vi "run_pharmaBotExp_v0.015.vi"(0 "data in":T12={"daq_ao 1"="Dev1/ao0", "daq_ai 1"="Dev1/ai0", "experiment day folder"=path "C:/multiBot/data/debug/testing", "Multiclamp init error"=0, "Multiclamp Handle Out"=10225184, "sampling rate (Hz)"=20000, "trial name"="t1"}, 1 "auto run?":bool=TRUE, 3 "which manipulator":T13(ring), 4 "HEK/slice options":enum16{"slice", "HEK"}(ring), 5 "error in":errorcluster, 6 "Validate after Experiment":bool, 7 "common cluster":T9, 11 "individual controls in":T8, 13 "images":T3={"slice image"="remote image 000000001461186C", "pipette template"="remote image 000000001461152C", "found pipette"=refnum, "pipette mask for cell tracker"=refnum, "cell images ref"=refnum}) -> (10 "Cell Looks Good?":bool=TRUE, 12 "ValidationOutputCluster":T5(array[cluster]), 14 "ValidationResults":waveform(dbl)[][](array[waveform]), 15 "ValidationPos1":T6(array[ring]), 16 "Exp. Terminated":bool, 17 "ValidationPos2":T6(array[ring]), 18 "ValidationWaveform":waveform(dbl)[](array[waveform]), 19 "error out":errorcluster)   [LabVIEW 2015] (continued)
              frame "Gap Free Iclamp" {
                n1665 = property class="TabCtl (strict)"(reference=w2342, "Value"=w2341) -> ()  [unwired: 1 in, 2 out]
                n1666 = property class="TabCtl (strict)"(reference=w2342, "Visible"=TRUE) -> ()  [unwired: 1 in, 2 out]
              }
              frame "Current Pulse" {
                n1667 = property class="TabCtl (strict)"(reference=w2345, "Value"=w2344) -> ()  [unwired: 1 in, 2 out]
                n1668 = property class="TabCtl (strict)"(reference=w2345, "Visible"=TRUE) -> ()  [unwired: 1 in, 2 out]
              }
              frame "Current Ramp" {
                n1669 = property class="TabCtl (strict)"(reference=w2348, "Value"=w2347) -> ()  [unwired: 1 in, 2 out]
                n1670 = property class="TabCtl (strict)"(reference=w2348, "Visible"=TRUE) -> ()  [unwired: 1 in, 2 out]
              }
              frame "Multi M. Jump" {
                n1671 = property class="TabCtl (strict)"(reference=w2351, "Value"=w2350) -> ()  [unwired: 1 in, 2 out]
                n1672 = property class="TabCtl (strict)"(reference=w2351, "Visible"=TRUE) -> ()  [unwired: 1 in, 2 out]
              }
              frame "none" {
                n1673 = property class="TabCtl (strict)"(reference=w2353, "Visible"=FALSE) -> ()  [unwired: 1 in, 2 out]
              }
            }
          }
          frame "PhaseL Experiment Option" {
            n1674 = control-ref of="Experiment Selection L"() -> (w2368:refnum<vi>)
            n1675 = case shown="\"Current Ramp\"" w2369 {
              tunnel: w2368 -> [_ w2371 w2374 w2377 w2380 w2383 w2386 w2389 w2392 w2395 w2398 w2401 w2404 w2407 w2409]
              tunnel: w2367 -> [_ _ _ _ _ _ _ _ _ _ _ _ _ w2406 _]
              tunnel: w2366 -> [_ w2370 _ _ _ _ _ _ _ _ _ _ _ _ _]
              tunnel: w2365 -> [_ _ w2373 _ _ _ _ _ _ _ _ _ _ _ _]
              tunnel: w2364 -> [_ _ _ w2376 _ _ _ _ _ _ _ _ _ _ _]
              tunnel: w2363 -> [_ _ _ _ w2379 _ _ _ _ _ _ _ _ _ _]
              tunnel: w2362 -> [_ _ _ _ _ w2382 _ _ _ _ _ _ _ _ _]
              tunnel: w2361 -> [_ _ _ _ _ _ w2385 _ _ _ _ _ _ _ _]
              tunnel: w2360 -> [_ _ _ _ _ _ _ w2388 _ _ _ _ _ _ _]
              tunnel: w2359 -> [_ _ _ _ _ _ _ _ w2391 _ _ _ _ _ _]
              tunnel: w2358 -> [_ _ _ _ _ _ _ _ _ w2394 _ _ _ _ _]
              tunnel: w2357 -> [_ _ _ _ _ _ _ _ _ _ w2397 _ _ _ _]
              tunnel: w2356 -> [_ _ _ _ _ _ _ _ _ _ _ w2400 _ _ _]
              tunnel: w2355 -> [_ _ _ _ _ _ _ _ _ _ _ _ w2403 _ _]
              frame "False", Default {
              }
              frame "Single Jump" {
                n1676 = property class="TabCtl (strict)"(reference=w2371, "Value"=w2370) -> ()  [unwired: 1 in, 2 out]
                n1677 = property class="TabCtl (strict)"(reference=w2371, "Visible"=TRUE) -> ()  [unwired: 1 in, 2 out]
              }
              frame "Solution Change" {
                n1678 = property class="TabCtl (strict)"(reference=w2374, "Visible"=TRUE) -> ()  [unwired: 1 in, 2 out]
                n1679 = property class="TabCtl (strict)"(reference=w2374, "Value"=w2373) -> ()  [unwired: 1 in, 2 out]
              }
              frame "Voltage Step" {
                n1680 = property class="TabCtl (strict)"(reference=w2377, "Value"=w2376) -> ()  [unwired: 1 in, 2 out]
                n1681 = property class="TabCtl (strict)"(reference=w2377, "Visible"=TRUE) -> ()  [unwired: 1 in, 2 out]
              }
              frame "Voltage Ramp" {
                n1682 = property class="TabCtl (strict)"(reference=w2380, "Value"=w2379) -> ()  [unwired: 1 in, 2 out]
                n1683 = property class="TabCtl (strict)"(reference=w2380, "Visible"=TRUE) -> ()  [unwired: 1 in, 2 out]
              }
              frame "Voltage Pulse" {
                n1684 = property class="TabCtl (strict)"(reference=w2383, "Value"=w2382) -> ()  [unwired: 1 in, 2 out]
                n1685 = property class="TabCtl (strict)"(reference=w2383, "Visible"=TRUE) -> ()  [unwired: 1 in, 2 out]
              }
              frame "Jump Train" {
                n1686 = property class="TabCtl (strict)"(reference=w2386, "Value"=w2385) -> ()  [unwired: 1 in, 2 out]
                n1687 = property class="TabCtl (strict)"(reference=w2386, "Visible"=TRUE) -> ()  [unwired: 1 in, 2 out]
              }
              frame "Paired Pulse" {
                n1688 = property class="TabCtl (strict)"(reference=w2389, "Value"=w2388) -> ()  [unwired: 1 in, 2 out]
                n1689 = property class="TabCtl (strict)"(reference=w2389, "Visible"=TRUE) -> ()  [unwired: 1 in, 2 out]
              }
              frame "Single Manip Jump" {
                n1690 = property class="TabCtl (strict)"(reference=w2392, "Value"=w2391) -> ()  [unwired: 1 in, 2 out]
                n1691 = property class="TabCtl (strict)"(reference=w2392, "Visible"=TRUE) -> ()  [unwired: 1 in, 2 out]
              }
              frame "Gap Free" {
                n1692 = property class="TabCtl (strict)"(reference=w2395, "Value"=w2394) -> ()  [unwired: 1 in, 2 out]
                n1693 = property class="TabCtl (strict)"(reference=w2395, "Visible"=TRUE) -> ()  [unwired: 1 in, 2 out]
              }
              frame "Gap Free Iclamp" {
                n1694 = property class="TabCtl (strict)"(reference=w2398, "Value"=w2397) -> ()  [unwired: 1 in, 2 out]
                n1695 = property class="TabCtl (strict)"(reference=w2398, "Visible"=TRUE) -> ()  [unwired: 1 in, 2 out]
              }
              frame "Current Pulse" {
                n1696 = property class="TabCtl (strict)"(reference=w2401, "Value"=w2400) -> ()  [unwired: 1 in, 2 out]
                n1697 = property class="TabCtl (strict)"(reference=w2401, "Visible"=TRUE) -> ()  [unwired: 1 in, 2 out]
              }
              frame "Current Ramp" {
                n1698 = property class="TabCtl (strict)"(reference=w2404, "Value"=w2403) -> ()  [unwired: 1 in, 2 out]
                n1699 = property class="TabCtl (strict)"(reference=w2404, "Visible"=TRUE) -> ()  [unwired: 1 in, 2 out]
              }
              frame "Multi M. Jump" {
                n1700 = property class="TabCtl (strict)"(reference=w2407, "Value"=w2406) -> ()  [unwired: 1 in, 2 out]
                n1701 = property class="TabCtl (strict)"(reference=w2407, "Visible"=TRUE) -> ()  [unwired: 1 in, 2 out]
              }
              frame "none" {
                n1702 = property class="TabCtl (strict)"(reference=w2409, "Visible"=FALSE) -> ()  [unwired: 1 in, 2 out]
              }
            }
          }
        }
      }
      event "How Many Experimental Phases?": Value Change {
        n1703 = event-data() -> ("NewVal"=w2412:i32)  [unwired: 1 in, 5 out]
        n1704 = case shown="12" w2412 {
          frame 0, Default {
          }
          frame 1 {
            n1705 = control-ref of="PhaseB Experiment Option"() -> (w2458:refnum<vi>)
            n1706 = control-ref of="PhaseF Experiment Option"() -> (w2440:refnum<vi>)
            n1707 = control-ref of="PhaseA Experiment Option"() -> (w2460:refnum<vi>)
            n1708 = control-ref of="PhaseD Experiment Option"() -> (w2448:refnum<vi>)
            n1709 = control-ref of="PhaseC Experiment Option"() -> (w2449:refnum<vi>)
            n1710 = control-ref of="PhaseE Experiment Option"() -> (w2441:refnum<vi>)
            n1711 = property class="CmbBox"(reference=w2460, "Visible"=TRUE) -> ()  [unwired: 1 in, 2 out]
            n1712 = property class="CmbBox"(reference=w2458, "Visible"=FALSE) -> ()  [unwired: 1 in, 2 out]
            n1713 = property class="CmbBox"(reference=w2440, "Visible"=FALSE) -> ()  [unwired: 1 in, 2 out]
            n1714 = property class="CmbBox"(reference=w2448, "Visible"=FALSE) -> ()  [unwired: 1 in, 2 out]
            n1715 = property class="CmbBox"(reference=w2449, "Visible"=FALSE) -> ()  [unwired: 1 in, 2 out]
            n1716 = property class="CmbBox"(reference=w2441, "Visible"=FALSE) -> ()  [unwired: 1 in, 2 out]
            n1717 = control-ref of="Experiment Selection B"() -> (w2455:refnum<vi>)
            n1718 = control-ref of="Experiment Selection F"() -> (w2437:refnum<vi>)
            n1719 = control-ref of="Experiment Selection D"() -> (w2445:refnum<vi>)
            n1720 = control-ref of="Experiment Selection A"() -> (w2453:refnum<vi>)
            n1721 = control-ref of="Experiment Selection C"() -> (w2452:refnum<vi>)
            n1722 = control-ref of="Experiment Selection E"() -> (w2444:refnum<vi>)
            n1723 = property class="TabCtl (strict)"(reference=w2455, "Visible"=FALSE) -> ()  [unwired: 1 in, 2 out]
            n1724 = property class="TabCtl (strict)"(reference=w2453, "Visible"=TRUE) -> ()  [unwired: 1 in, 2 out]
            n1725 = property class="TabCtl (strict)"(reference=w2437, "Visible"=FALSE) -> ()  [unwired: 1 in, 2 out]
            n1726 = property class="TabCtl (strict)"(reference=w2445, "Visible"=FALSE) -> ()  [unwired: 1 in, 2 out]
            n1727 = property class="TabCtl (strict)"(reference=w2452, "Visible"=FALSE) -> ()  [unwired: 1 in, 2 out]
            n1728 = property class="TabCtl (strict)"(reference=w2444, "Visible"=FALSE) -> ()  [unwired: 1 in, 2 out]
            n1729 = control-ref of="PhaseH Experiment Option"() -> (w2415:refnum<vi>)
            n1730 = control-ref of="PhaseL Experiment Option"() -> (w2433:refnum<vi>)
            n1731 = control-ref of="PhaseG Experiment Option"() -> (w2413:refnum<vi>)
            n1732 = control-ref of="PhaseJ Experiment Option"() -> (w2425:refnum<vi>)
            n1733 = control-ref of="PhaseI Experiment Option"() -> (w2424:refnum<vi>)
            n1734 = control-ref of="PhaseK Experiment Option"() -> (w2432:refnum<vi>)
            n1735 = property class="CmbBox"(reference=w2413, "Visible"=FALSE) -> ()  [unwired: 1 in, 2 out]
            n1736 = property class="CmbBox"(reference=w2415, "Visible"=FALSE) -> ()  [unwired: 1 in, 2 out]
            n1737 = property class="CmbBox"(reference=w2433, "Visible"=FALSE) -> ()  [unwired: 1 in, 2 out]
            n1738 = property class="CmbBox"(reference=w2425, "Visible"=FALSE) -> ()  [unwired: 1 in, 2 out]
            n1739 = property class="CmbBox"(reference=w2424, "Visible"=FALSE) -> ()  [unwired: 1 in, 2 out]
            n1740 = property class="CmbBox"(reference=w2432, "Visible"=FALSE) -> ()  [unwired: 1 in, 2 out]
            n1741 = control-ref of="Experiment Selection H"() -> (w2418:refnum<vi>)
            n1742 = control-ref of="Experiment Selection L"() -> (w2436:refnum<vi>)
            n1743 = control-ref of="Experiment Selection J"() -> (w2428:refnum<vi>)
            n1744 = control-ref of="Experiment Selection G"() -> (w2420:refnum<vi>)
            n1745 = control-ref of="Experiment Selection I"() -> (w2421:refnum<vi>)
            n1746 = control-ref of="Experiment Selection K"() -> (w2429:refnum<vi>)
            n1747 = property class="TabCtl (strict)"(reference=w2418, "Visible"=FALSE) -> ()  [unwired: 1 in, 2 out]
            n1748 = property class="TabCtl (strict)"(reference=w2420, "Visible"=FALSE) -> ()  [unwired: 1 in, 2 out]
            n1749 = property class="TabCtl (strict)"(reference=w2436, "Visible"=FALSE) -> ()  [unwired: 1 in, 2 out]
            n1750 = property class="TabCtl (strict)"(reference=w2428, "Visible"=FALSE) -> ()  [unwired: 1 in, 2 out]
            n1751 = property class="TabCtl (strict)"(reference=w2421, "Visible"=FALSE) -> ()  [unwired: 1 in, 2 out]
            n1752 = property class="TabCtl (strict)"(reference=w2429, "Visible"=FALSE) -> ()  [unwired: 1 in, 2 out]
          }
          frame 2 {
            n1753 = control-ref of="PhaseB Experiment Option"() -> (w2506:refnum<vi>)
            n1754 = control-ref of="PhaseF Experiment Option"() -> (w2488:refnum<vi>)
            n1755 = control-ref of="PhaseA Experiment Option"() -> (w2508:refnum<vi>)
            n1756 = control-ref of="PhaseD Experiment Option"() -> (w2496:refnum<vi>)
            n1757 = control-ref of="PhaseC Experiment Option"() -> (w2497:refnum<vi>)
            n1758 = control-ref of="PhaseE Experiment Option"() -> (w2489:refnum<vi>)
            n1759 = property class="CmbBox"(reference=w2508, "Visible"=TRUE) -> ()  [unwired: 1 in, 2 out]
            n1760 = property class="CmbBox"(reference=w2506, "Visible"=TRUE) -> ()  [unwired: 1 in, 2 out]
            n1761 = property class="CmbBox"(reference=w2488, "Visible"=FALSE) -> ()  [unwired: 1 in, 2 out]
            n1762 = property class="CmbBox"(reference=w2496, "Visible"=FALSE) -> ()  [unwired: 1 in, 2 out]
            n1763 = property class="CmbBox"(reference=w2497, "Visible"=FALSE) -> ()  [unwired: 1 in, 2 out]
            n1764 = property class="CmbBox"(reference=w2489, "Visible"=FALSE) -> ()  [unwired: 1 in, 2 out]
            n1765 = control-ref of="Experiment Selection B"() -> (w2503:refnum<vi>)
            n1766 = control-ref of="Experiment Selection F"() -> (w2485:refnum<vi>)
            n1767 = control-ref of="Experiment Selection D"() -> (w2493:refnum<vi>)
            n1768 = control-ref of="Experiment Selection A"() -> (w2501:refnum<vi>)
            n1769 = control-ref of="Experiment Selection C"() -> (w2500:refnum<vi>)
            n1770 = control-ref of="Experiment Selection E"() -> (w2492:refnum<vi>)
            n1771 = property class="TabCtl (strict)"(reference=w2503, "Visible"=TRUE) -> ()  [unwired: 1 in, 2 out]
            n1772 = property class="TabCtl (strict)"(reference=w2501, "Visible"=TRUE) -> ()  [unwired: 1 in, 2 out]
            n1773 = property class="TabCtl (strict)"(reference=w2485, "Visible"=FALSE) -> ()  [unwired: 1 in, 2 out]
            n1774 = property class="TabCtl (strict)"(reference=w2493, "Visible"=FALSE) -> ()  [unwired: 1 in, 2 out]
            n1775 = property class="TabCtl (strict)"(reference=w2500, "Visible"=FALSE) -> ()  [unwired: 1 in, 2 out]
            n1776 = property class="TabCtl (strict)"(reference=w2492, "Visible"=FALSE) -> ()  [unwired: 1 in, 2 out]
            n1777 = control-ref of="PhaseH Experiment Option"() -> (w2463:refnum<vi>)
            n1778 = control-ref of="PhaseL Experiment Option"() -> (w2481:refnum<vi>)
            n1779 = control-ref of="PhaseG Experiment Option"() -> (w2461:refnum<vi>)
            n1780 = control-ref of="PhaseJ Experiment Option"() -> (w2473:refnum<vi>)
            n1781 = control-ref of="PhaseI Experiment Option"() -> (w2472:refnum<vi>)
            n1782 = control-ref of="PhaseK Experiment Option"() -> (w2480:refnum<vi>)
            n1783 = property class="CmbBox"(reference=w2461, "Visible"=FALSE) -> ()  [unwired: 1 in, 2 out]
            n1784 = property class="CmbBox"(reference=w2463, "Visible"=FALSE) -> ()  [unwired: 1 in, 2 out]
            n1785 = property class="CmbBox"(reference=w2481, "Visible"=FALSE) -> ()  [unwired: 1 in, 2 out]
            n1786 = property class="CmbBox"(reference=w2473, "Visible"=FALSE) -> ()  [unwired: 1 in, 2 out]
            n1787 = property class="CmbBox"(reference=w2472, "Visible"=FALSE) -> ()  [unwired: 1 in, 2 out]
            n1788 = property class="CmbBox"(reference=w2480, "Visible"=FALSE) -> ()  [unwired: 1 in, 2 out]
            n1789 = control-ref of="Experiment Selection H"() -> (w2466:refnum<vi>)
            n1790 = control-ref of="Experiment Selection L"() -> (w2484:refnum<vi>)
            n1791 = control-ref of="Experiment Selection J"() -> (w2476:refnum<vi>)
            n1792 = control-ref of="Experiment Selection G"() -> (w2468:refnum<vi>)
            n1793 = control-ref of="Experiment Selection I"() -> (w2469:refnum<vi>)
            n1794 = control-ref of="Experiment Selection K"() -> (w2477:refnum<vi>)
            n1795 = property class="TabCtl (strict)"(reference=w2466, "Visible"=FALSE) -> ()  [unwired: 1 in, 2 out]
            n1796 = property class="TabCtl (strict)"(reference=w2468, "Visible"=FALSE) -> ()  [unwired: 1 in, 2 out]
            n1797 = property class="TabCtl (strict)"(reference=w2484, "Visible"=FALSE) -> ()  [unwired: 1 in, 2 out]
            n1798 = property class="TabCtl (strict)"(reference=w2476, "Visible"=FALSE) -> ()  [unwired: 1 in, 2 out]
            n1799 = property class="TabCtl (strict)"(reference=w2469, "Visible"=FALSE) -> ()  [unwired: 1 in, 2 out]
            n1800 = property class="TabCtl (strict)"(reference=w2477, "Visible"=FALSE) -> ()  [unwired: 1 in, 2 out]
          }
          frame 3 {
            n1801 = control-ref of="PhaseB Experiment Option"() -> (w2554:refnum<vi>)
            n1802 = control-ref of="PhaseF Experiment Option"() -> (w2536:refnum<vi>)
            n1803 = control-ref of="PhaseA Experiment Option"() -> (w2556:refnum<vi>)
            n1804 = control-ref of="PhaseD Experiment Option"() -> (w2544:refnum<vi>)
            n1805 = control-ref of="PhaseC Experiment Option"() -> (w2545:refnum<vi>)
            n1806 = control-ref of="PhaseE Experiment Option"() -> (w2537:refnum<vi>)
            n1807 = property class="CmbBox"(reference=w2556, "Visible"=TRUE) -> ()  [unwired: 1 in, 2 out]
            n1808 = property class="CmbBox"(reference=w2554, "Visible"=TRUE) -> ()  [unwired: 1 in, 2 out]
            n1809 = property class="CmbBox"(reference=w2536, "Visible"=FALSE) -> ()  [unwired: 1 in, 2 out]
            n1810 = property class="CmbBox"(reference=w2544, "Visible"=FALSE) -> ()  [unwired: 1 in, 2 out]
            n1811 = property class="CmbBox"(reference=w2545, "Visible"=TRUE) -> ()  [unwired: 1 in, 2 out]
            n1812 = property class="CmbBox"(reference=w2537, "Visible"=FALSE) -> ()  [unwired: 1 in, 2 out]
            n1813 = control-ref of="Experiment Selection B"() -> (w2551:refnum<vi>)
            n1814 = control-ref of="Experiment Selection F"() -> (w2533:refnum<vi>)
            n1815 = control-ref of="Experiment Selection D"() -> (w2541:refnum<vi>)
            n1816 = control-ref of="Experiment Selection A"() -> (w2549:refnum<vi>)
            n1817 = control-ref of="Experiment Selection C"() -> (w2548:refnum<vi>)
            n1818 = control-ref of="Experiment Selection E"() -> (w2540:refnum<vi>)
            n1819 = property class="TabCtl (strict)"(reference=w2551, "Visible"=TRUE) -> ()  [unwired: 1 in, 2 out]
            n1820 = property class="TabCtl (strict)"(reference=w2549, "Visible"=TRUE) -> ()  [unwired: 1 in, 2 out]
            n1821 = property class="TabCtl (strict)"(reference=w2533, "Visible"=FALSE) -> ()  [unwired: 1 in, 2 out]
            n1822 = property class="TabCtl (strict)"(reference=w2541, "Visible"=FALSE) -> ()  [unwired: 1 in, 2 out]
            n1823 = property class="TabCtl (strict)"(reference=w2548, "Visible"=TRUE) -> ()  [unwired: 1 in, 2 out]
            n1824 = property class="TabCtl (strict)"(reference=w2540, "Visible"=FALSE) -> ()  [unwired: 1 in, 2 out]
            n1825 = control-ref of="PhaseH Experiment Option"() -> (w2511:refnum<vi>)
            n1826 = control-ref of="PhaseL Experiment Option"() -> (w2529:refnum<vi>)
            n1827 = control-ref of="PhaseG Experiment Option"() -> (w2509:refnum<vi>)
            n1828 = control-ref of="PhaseJ Experiment Option"() -> (w2521:refnum<vi>)
            n1829 = control-ref of="PhaseI Experiment Option"() -> (w2520:refnum<vi>)
            n1830 = control-ref of="PhaseK Experiment Option"() -> (w2528:refnum<vi>)
            n1831 = property class="CmbBox"(reference=w2509, "Visible"=FALSE) -> ()  [unwired: 1 in, 2 out]
            n1832 = property class="CmbBox"(reference=w2511, "Visible"=FALSE) -> ()  [unwired: 1 in, 2 out]
            n1833 = property class="CmbBox"(reference=w2529, "Visible"=FALSE) -> ()  [unwired: 1 in, 2 out]
            n1834 = property class="CmbBox"(reference=w2521, "Visible"=FALSE) -> ()  [unwired: 1 in, 2 out]
            n1835 = property class="CmbBox"(reference=w2520, "Visible"=FALSE) -> ()  [unwired: 1 in, 2 out]
            n1836 = property class="CmbBox"(reference=w2528, "Visible"=FALSE) -> ()  [unwired: 1 in, 2 out]
            n1837 = control-ref of="Experiment Selection H"() -> (w2514:refnum<vi>)
            n1838 = control-ref of="Experiment Selection L"() -> (w2532:refnum<vi>)
            n1839 = control-ref of="Experiment Selection J"() -> (w2524:refnum<vi>)
            n1840 = control-ref of="Experiment Selection G"() -> (w2516:refnum<vi>)
            n1841 = control-ref of="Experiment Selection I"() -> (w2517:refnum<vi>)
            n1842 = control-ref of="Experiment Selection K"() -> (w2525:refnum<vi>)
            n1843 = property class="TabCtl (strict)"(reference=w2514, "Visible"=FALSE) -> ()  [unwired: 1 in, 2 out]
            n1844 = property class="TabCtl (strict)"(reference=w2516, "Visible"=FALSE) -> ()  [unwired: 1 in, 2 out]
            n1845 = property class="TabCtl (strict)"(reference=w2532, "Visible"=FALSE) -> ()  [unwired: 1 in, 2 out]
            n1846 = property class="TabCtl (strict)"(reference=w2524, "Visible"=FALSE) -> ()  [unwired: 1 in, 2 out]
            n1847 = property class="TabCtl (strict)"(reference=w2517, "Visible"=FALSE) -> ()  [unwired: 1 in, 2 out]
            n1848 = property class="TabCtl (strict)"(reference=w2525, "Visible"=FALSE) -> ()  [unwired: 1 in, 2 out]
          }
          frame 4 {
            n1849 = control-ref of="PhaseB Experiment Option"() -> (w2602:refnum<vi>)
            n1850 = control-ref of="PhaseF Experiment Option"() -> (w2584:refnum<vi>)
            n1851 = control-ref of="PhaseA Experiment Option"() -> (w2604:refnum<vi>)
            n1852 = control-ref of="PhaseD Experiment Option"() -> (w2592:refnum<vi>)
            n1853 = control-ref of="PhaseC Experiment Option"() -> (w2593:refnum<vi>)
            n1854 = control-ref of="PhaseE Experiment Option"() -> (w2585:refnum<vi>)
            n1855 = property class="CmbBox"(reference=w2604, "Visible"=TRUE) -> ()  [unwired: 1 in, 2 out]
            n1856 = property class="CmbBox"(reference=w2602, "Visible"=TRUE) -> ()  [unwired: 1 in, 2 out]
            n1857 = property class="CmbBox"(reference=w2584, "Visible"=FALSE) -> ()  [unwired: 1 in, 2 out]
            n1858 = property class="CmbBox"(reference=w2592, "Visible"=TRUE) -> ()  [unwired: 1 in, 2 out]
            n1859 = property class="CmbBox"(reference=w2593, "Visible"=TRUE) -> ()  [unwired: 1 in, 2 out]
            n1860 = property class="CmbBox"(reference=w2585, "Visible"=FALSE) -> ()  [unwired: 1 in, 2 out]
            n1861 = control-ref of="Experiment Selection B"() -> (w2599:refnum<vi>)
            n1862 = control-ref of="Experiment Selection F"() -> (w2581:refnum<vi>)
            n1863 = control-ref of="Experiment Selection D"() -> (w2589:refnum<vi>)
            n1864 = control-ref of="Experiment Selection A"() -> (w2597:refnum<vi>)
            n1865 = control-ref of="Experiment Selection C"() -> (w2596:refnum<vi>)
            n1866 = control-ref of="Experiment Selection E"() -> (w2588:refnum<vi>)
            n1867 = property class="TabCtl (strict)"(reference=w2599, "Visible"=TRUE) -> ()  [unwired: 1 in, 2 out]
            n1868 = property class="TabCtl (strict)"(reference=w2597, "Visible"=TRUE) -> ()  [unwired: 1 in, 2 out]
            n1869 = property class="TabCtl (strict)"(reference=w2581, "Visible"=FALSE) -> ()  [unwired: 1 in, 2 out]
            n1870 = property class="TabCtl (strict)"(reference=w2589, "Visible"=TRUE) -> ()  [unwired: 1 in, 2 out]
            n1871 = property class="TabCtl (strict)"(reference=w2596, "Visible"=TRUE) -> ()  [unwired: 1 in, 2 out]
            n1872 = property class="TabCtl (strict)"(reference=w2588, "Visible"=FALSE) -> ()  [unwired: 1 in, 2 out]
            n1873 = control-ref of="PhaseH Experiment Option"() -> (w2559:refnum<vi>)
            n1874 = control-ref of="PhaseL Experiment Option"() -> (w2577:refnum<vi>)
            n1875 = control-ref of="PhaseG Experiment Option"() -> (w2557:refnum<vi>)
            n1876 = control-ref of="PhaseJ Experiment Option"() -> (w2569:refnum<vi>)
            n1877 = control-ref of="PhaseI Experiment Option"() -> (w2568:refnum<vi>)
            n1878 = control-ref of="PhaseK Experiment Option"() -> (w2576:refnum<vi>)
            n1879 = property class="CmbBox"(reference=w2557, "Visible"=FALSE) -> ()  [unwired: 1 in, 2 out]
            n1880 = property class="CmbBox"(reference=w2559, "Visible"=FALSE) -> ()  [unwired: 1 in, 2 out]
            n1881 = property class="CmbBox"(reference=w2577, "Visible"=FALSE) -> ()  [unwired: 1 in, 2 out]
            n1882 = property class="CmbBox"(reference=w2569, "Visible"=FALSE) -> ()  [unwired: 1 in, 2 out]
            n1883 = property class="CmbBox"(reference=w2568, "Visible"=FALSE) -> ()  [unwired: 1 in, 2 out]
            n1884 = property class="CmbBox"(reference=w2576, "Visible"=FALSE) -> ()  [unwired: 1 in, 2 out]
            n1885 = control-ref of="Experiment Selection H"() -> (w2562:refnum<vi>)
            n1886 = control-ref of="Experiment Selection L"() -> (w2580:refnum<vi>)
            n1887 = control-ref of="Experiment Selection J"() -> (w2572:refnum<vi>)
            n1888 = control-ref of="Experiment Selection G"() -> (w2564:refnum<vi>)
            n1889 = control-ref of="Experiment Selection I"() -> (w2565:refnum<vi>)
            n1890 = control-ref of="Experiment Selection K"() -> (w2573:refnum<vi>)
            n1891 = property class="TabCtl (strict)"(reference=w2562, "Visible"=FALSE) -> ()  [unwired: 1 in, 2 out]
            n1892 = property class="TabCtl (strict)"(reference=w2564, "Visible"=FALSE) -> ()  [unwired: 1 in, 2 out]
            n1893 = property class="TabCtl (strict)"(reference=w2580, "Visible"=FALSE) -> ()  [unwired: 1 in, 2 out]
            n1894 = property class="TabCtl (strict)"(reference=w2572, "Visible"=FALSE) -> ()  [unwired: 1 in, 2 out]
            n1895 = property class="TabCtl (strict)"(reference=w2565, "Visible"=FALSE) -> ()  [unwired: 1 in, 2 out]
            n1896 = property class="TabCtl (strict)"(reference=w2573, "Visible"=FALSE) -> ()  [unwired: 1 in, 2 out]
          }
          frame 5 {
            n1897 = control-ref of="PhaseB Experiment Option"() -> (w2650:refnum<vi>)
            n1898 = control-ref of="PhaseF Experiment Option"() -> (w2632:refnum<vi>)
            n1899 = control-ref of="PhaseA Experiment Option"() -> (w2652:refnum<vi>)
            n1900 = control-ref of="PhaseD Experiment Option"() -> (w2640:refnum<vi>)
            n1901 = control-ref of="PhaseC Experiment Option"() -> (w2641:refnum<vi>)
            n1902 = control-ref of="PhaseE Experiment Option"() -> (w2633:refnum<vi>)
            n1903 = property class="CmbBox"(reference=w2652, "Visible"=TRUE) -> ()  [unwired: 1 in, 2 out]
            n1904 = property class="CmbBox"(reference=w2650, "Visible"=TRUE) -> ()  [unwired: 1 in, 2 out]
            n1905 = property class="CmbBox"(reference=w2632, "Visible"=FALSE) -> ()  [unwired: 1 in, 2 out]
            n1906 = property class="CmbBox"(reference=w2640, "Visible"=TRUE) -> ()  [unwired: 1 in, 2 out]
            n1907 = property class="CmbBox"(reference=w2641, "Visible"=TRUE) -> ()  [unwired: 1 in, 2 out]
            n1908 = property class="CmbBox"(reference=w2633, "Visible"=TRUE) -> ()  [unwired: 1 in, 2 out]
            n1909 = control-ref of="Experiment Selection B"() -> (w2647:refnum<vi>)
            n1910 = control-ref of="Experiment Selection F"() -> (w2629:refnum<vi>)
            n1911 = control-ref of="Experiment Selection D"() -> (w2637:refnum<vi>)
            n1912 = control-ref of="Experiment Selection A"() -> (w2645:refnum<vi>)
            n1913 = control-ref of="Experiment Selection C"() -> (w2644:refnum<vi>)
            n1914 = control-ref of="Experiment Selection E"() -> (w2636:refnum<vi>)
            n1915 = property class="TabCtl (strict)"(reference=w2647, "Visible"=TRUE) -> ()  [unwired: 1 in, 2 out]
            n1916 = property class="TabCtl (strict)"(reference=w2645, "Visible"=TRUE) -> ()  [unwired: 1 in, 2 out]
            n1917 = property class="TabCtl (strict)"(reference=w2629, "Visible"=FALSE) -> ()  [unwired: 1 in, 2 out]
            n1918 = property class="TabCtl (strict)"(reference=w2637, "Visible"=TRUE) -> ()  [unwired: 1 in, 2 out]
            n1919 = property class="TabCtl (strict)"(reference=w2644, "Visible"=TRUE) -> ()  [unwired: 1 in, 2 out]
            n1920 = property class="TabCtl (strict)"(reference=w2636, "Visible"=TRUE) -> ()  [unwired: 1 in, 2 out]
            n1921 = control-ref of="PhaseH Experiment Option"() -> (w2607:refnum<vi>)
            n1922 = control-ref of="PhaseL Experiment Option"() -> (w2625:refnum<vi>)
            n1923 = control-ref of="PhaseG Experiment Option"() -> (w2605:refnum<vi>)
            n1924 = control-ref of="PhaseJ Experiment Option"() -> (w2617:refnum<vi>)
            n1925 = control-ref of="PhaseI Experiment Option"() -> (w2616:refnum<vi>)
            n1926 = control-ref of="PhaseK Experiment Option"() -> (w2624:refnum<vi>)
            n1927 = property class="CmbBox"(reference=w2605, "Visible"=FALSE) -> ()  [unwired: 1 in, 2 out]
            n1928 = property class="CmbBox"(reference=w2607, "Visible"=FALSE) -> ()  [unwired: 1 in, 2 out]
            n1929 = property class="CmbBox"(reference=w2625, "Visible"=FALSE) -> ()  [unwired: 1 in, 2 out]
            n1930 = property class="CmbBox"(reference=w2617, "Visible"=FALSE) -> ()  [unwired: 1 in, 2 out]
            n1931 = property class="CmbBox"(reference=w2616, "Visible"=FALSE) -> ()  [unwired: 1 in, 2 out]
            n1932 = property class="CmbBox"(reference=w2624, "Visible"=FALSE) -> ()  [unwired: 1 in, 2 out]
            n1933 = control-ref of="Experiment Selection H"() -> (w2610:refnum<vi>)
            n1934 = control-ref of="Experiment Selection L"() -> (w2628:refnum<vi>)
            n1935 = control-ref of="Experiment Selection J"() -> (w2620:refnum<vi>)
            n1936 = control-ref of="Experiment Selection G"() -> (w2612:refnum<vi>)
            n1937 = control-ref of="Experiment Selection I"() -> (w2613:refnum<vi>)
            n1938 = control-ref of="Experiment Selection K"() -> (w2621:refnum<vi>)
            n1939 = property class="TabCtl (strict)"(reference=w2610, "Visible"=FALSE) -> ()  [unwired: 1 in, 2 out]
            n1940 = property class="TabCtl (strict)"(reference=w2612, "Visible"=FALSE) -> ()  [unwired: 1 in, 2 out]
            n1941 = property class="TabCtl (strict)"(reference=w2628, "Visible"=FALSE) -> ()  [unwired: 1 in, 2 out]
            n1942 = property class="TabCtl (strict)"(reference=w2620, "Visible"=FALSE) -> ()  [unwired: 1 in, 2 out]
            n1943 = property class="TabCtl (strict)"(reference=w2613, "Visible"=FALSE) -> ()  [unwired: 1 in, 2 out]
            n1944 = property class="TabCtl (strict)"(reference=w2621, "Visible"=FALSE) -> ()  [unwired: 1 in, 2 out]
          }
          frame 6 {
            n1945 = control-ref of="PhaseB Experiment Option"() -> (w2698:refnum<vi>)
            n1946 = control-ref of="PhaseF Experiment Option"() -> (w2680:refnum<vi>)
            n1947 = control-ref of="PhaseA Experiment Option"() -> (w2700:refnum<vi>)
            n1948 = control-ref of="PhaseD Experiment Option"() -> (w2688:refnum<vi>)
            n1949 = control-ref of="PhaseC Experiment Option"() -> (w2689:refnum<vi>)
            n1950 = control-ref of="PhaseE Experiment Option"() -> (w2681:refnum<vi>)
            n1951 = property class="CmbBox"(reference=w2700, "Visible"=TRUE) -> ()  [unwired: 1 in, 2 out]
            n1952 = property class="CmbBox"(reference=w2698, "Visible"=TRUE) -> ()  [unwired: 1 in, 2 out]
            n1953 = property class="CmbBox"(reference=w2680, "Visible"=TRUE) -> ()  [unwired: 1 in, 2 out]
            n1954 = property class="CmbBox"(reference=w2688, "Visible"=TRUE) -> ()  [unwired: 1 in, 2 out]
            n1955 = property class="CmbBox"(reference=w2689, "Visible"=TRUE) -> ()  [unwired: 1 in, 2 out]
            n1956 = property class="CmbBox"(reference=w2681, "Visible"=TRUE) -> ()  [unwired: 1 in, 2 out]
            n1957 = control-ref of="Experiment Selection B"() -> (w2695:refnum<vi>)
            n1958 = control-ref of="Experiment Selection F"() -> (w2677:refnum<vi>)
            n1959 = control-ref of="Experiment Selection D"() -> (w2685:refnum<vi>)
            n1960 = control-ref of="Experiment Selection A"() -> (w2693:refnum<vi>)
            n1961 = control-ref of="Experiment Selection C"() -> (w2692:refnum<vi>)
            n1962 = control-ref of="Experiment Selection E"() -> (w2684:refnum<vi>)
            n1963 = property class="TabCtl (strict)"(reference=w2695, "Visible"=TRUE) -> ()  [unwired: 1 in, 2 out]
            n1964 = property class="TabCtl (strict)"(reference=w2693, "Visible"=TRUE) -> ()  [unwired: 1 in, 2 out]
            n1965 = property class="TabCtl (strict)"(reference=w2677, "Visible"=TRUE) -> ()  [unwired: 1 in, 2 out]
            n1966 = property class="TabCtl (strict)"(reference=w2685, "Visible"=TRUE) -> ()  [unwired: 1 in, 2 out]
            n1967 = property class="TabCtl (strict)"(reference=w2692, "Visible"=TRUE) -> ()  [unwired: 1 in, 2 out]
            n1968 = property class="TabCtl (strict)"(reference=w2684, "Visible"=TRUE) -> ()  [unwired: 1 in, 2 out]
            n1969 = control-ref of="PhaseH Experiment Option"() -> (w2655:refnum<vi>)
            n1970 = control-ref of="PhaseL Experiment Option"() -> (w2673:refnum<vi>)
            n1971 = control-ref of="PhaseG Experiment Option"() -> (w2653:refnum<vi>)
            n1972 = control-ref of="PhaseJ Experiment Option"() -> (w2665:refnum<vi>)
            n1973 = control-ref of="PhaseI Experiment Option"() -> (w2664:refnum<vi>)
            n1974 = control-ref of="PhaseK Experiment Option"() -> (w2672:refnum<vi>)
            n1975 = property class="CmbBox"(reference=w2653, "Visible"=FALSE) -> ()  [unwired: 1 in, 2 out]
            n1976 = property class="CmbBox"(reference=w2655, "Visible"=FALSE) -> ()  [unwired: 1 in, 2 out]
            n1977 = property class="CmbBox"(reference=w2673, "Visible"=FALSE) -> ()  [unwired: 1 in, 2 out]
            n1978 = property class="CmbBox"(reference=w2665, "Visible"=FALSE) -> ()  [unwired: 1 in, 2 out]
            n1979 = property class="CmbBox"(reference=w2664, "Visible"=FALSE) -> ()  [unwired: 1 in, 2 out]
            n1980 = property class="CmbBox"(reference=w2672, "Visible"=FALSE) -> ()  [unwired: 1 in, 2 out]
            n1981 = control-ref of="Experiment Selection H"() -> (w2658:refnum<vi>)
            n1982 = control-ref of="Experiment Selection L"() -> (w2676:refnum<vi>)
            n1983 = control-ref of="Experiment Selection J"() -> (w2668:refnum<vi>)
            n1984 = control-ref of="Experiment Selection G"() -> (w2660:refnum<vi>)
            n1985 = control-ref of="Experiment Selection I"() -> (w2661:refnum<vi>)
            n1986 = control-ref of="Experiment Selection K"() -> (w2669:refnum<vi>)
            n1987 = property class="TabCtl (strict)"(reference=w2658, "Visible"=FALSE) -> ()  [unwired: 1 in, 2 out]
            n1988 = property class="TabCtl (strict)"(reference=w2660, "Visible"=FALSE) -> ()  [unwired: 1 in, 2 out]
            n1989 = property class="TabCtl (strict)"(reference=w2676, "Visible"=FALSE) -> ()  [unwired: 1 in, 2 out]
            n1990 = property class="TabCtl (strict)"(reference=w2668, "Visible"=FALSE) -> ()  [unwired: 1 in, 2 out]
            n1991 = property class="TabCtl (strict)"(reference=w2661, "Visible"=FALSE) -> ()  [unwired: 1 in, 2 out]
            n1992 = property class="TabCtl (strict)"(reference=w2669, "Visible"=FALSE) -> ()  [unwired: 1 in, 2 out]
          }
          frame 7 {
            n1993 = control-ref of="PhaseB Experiment Option"() -> (w2746:refnum<vi>)
            n1994 = control-ref of="PhaseF Experiment Option"() -> (w2728:refnum<vi>)
            n1995 = control-ref of="PhaseA Experiment Option"() -> (w2748:refnum<vi>)
            n1996 = control-ref of="PhaseD Experiment Option"() -> (w2736:refnum<vi>)
            n1997 = control-ref of="PhaseC Experiment Option"() -> (w2737:refnum<vi>)
            n1998 = control-ref of="PhaseE Experiment Option"() -> (w2729:refnum<vi>)
            n1999 = property class="CmbBox"(reference=w2748, "Visible"=TRUE) -> ()  [unwired: 1 in, 2 out]
            n2000 = property class="CmbBox"(reference=w2746, "Visible"=TRUE) -> ()  [unwired: 1 in, 2 out]
            n2001 = property class="CmbBox"(reference=w2728, "Visible"=TRUE) -> ()  [unwired: 1 in, 2 out]
            n2002 = property class="CmbBox"(reference=w2736, "Visible"=TRUE) -> ()  [unwired: 1 in, 2 out]
            n2003 = property class="CmbBox"(reference=w2737, "Visible"=TRUE) -> ()  [unwired: 1 in, 2 out]
            n2004 = property class="CmbBox"(reference=w2729, "Visible"=TRUE) -> ()  [unwired: 1 in, 2 out]
            n2005 = control-ref of="Experiment Selection B"() -> (w2743:refnum<vi>)
            n2006 = control-ref of="Experiment Selection F"() -> (w2725:refnum<vi>)
            n2007 = control-ref of="Experiment Selection D"() -> (w2733:refnum<vi>)
            n2008 = control-ref of="Experiment Selection A"() -> (w2741:refnum<vi>)
            n2009 = control-ref of="Experiment Selection C"() -> (w2740:refnum<vi>)
            n2010 = control-ref of="Experiment Selection E"() -> (w2732:refnum<vi>)
            n2011 = property class="TabCtl (strict)"(reference=w2743, "Visible"=TRUE) -> ()  [unwired: 1 in, 2 out]
            n2012 = property class="TabCtl (strict)"(reference=w2741, "Visible"=TRUE) -> ()  [unwired: 1 in, 2 out]
            n2013 = property class="TabCtl (strict)"(reference=w2725, "Visible"=TRUE) -> ()  [unwired: 1 in, 2 out]
            n2014 = property class="TabCtl (strict)"(reference=w2733, "Visible"=TRUE) -> ()  [unwired: 1 in, 2 out]
            n2015 = property class="TabCtl (strict)"(reference=w2740, "Visible"=TRUE) -> ()  [unwired: 1 in, 2 out]
            n2016 = property class="TabCtl (strict)"(reference=w2732, "Visible"=TRUE) -> ()  [unwired: 1 in, 2 out]
            n2017 = control-ref of="PhaseH Experiment Option"() -> (w2703:refnum<vi>)
            n2018 = control-ref of="PhaseL Experiment Option"() -> (w2721:refnum<vi>)
            n2019 = control-ref of="PhaseG Experiment Option"() -> (w2701:refnum<vi>)
            n2020 = control-ref of="PhaseJ Experiment Option"() -> (w2713:refnum<vi>)
            n2021 = control-ref of="PhaseI Experiment Option"() -> (w2712:refnum<vi>)
            n2022 = control-ref of="PhaseK Experiment Option"() -> (w2720:refnum<vi>)
            n2023 = property class="CmbBox"(reference=w2701, "Visible"=TRUE) -> ()  [unwired: 1 in, 2 out]
            n2024 = property class="CmbBox"(reference=w2703, "Visible"=FALSE) -> ()  [unwired: 1 in, 2 out]
            n2025 = property class="CmbBox"(reference=w2721, "Visible"=FALSE) -> ()  [unwired: 1 in, 2 out]
            n2026 = property class="CmbBox"(reference=w2713, "Visible"=FALSE) -> ()  [unwired: 1 in, 2 out]
            n2027 = property class="CmbBox"(reference=w2712, "Visible"=FALSE) -> ()  [unwired: 1 in, 2 out]
            n2028 = property class="CmbBox"(reference=w2720, "Visible"=FALSE) -> ()  [unwired: 1 in, 2 out]
            n2029 = control-ref of="Experiment Selection H"() -> (w2706:refnum<vi>)
            n2030 = control-ref of="Experiment Selection L"() -> (w2724:refnum<vi>)
            n2031 = control-ref of="Experiment Selection J"() -> (w2716:refnum<vi>)
            n2032 = control-ref of="Experiment Selection G"() -> (w2708:refnum<vi>)
            n2033 = control-ref of="Experiment Selection I"() -> (w2709:refnum<vi>)
            n2034 = control-ref of="Experiment Selection K"() -> (w2717:refnum<vi>)
            n2035 = property class="TabCtl (strict)"(reference=w2706, "Visible"=FALSE) -> ()  [unwired: 1 in, 2 out]
            n2036 = property class="TabCtl (strict)"(reference=w2708, "Visible"=TRUE) -> ()  [unwired: 1 in, 2 out]
            n2037 = property class="TabCtl (strict)"(reference=w2724, "Visible"=FALSE) -> ()  [unwired: 1 in, 2 out]
            n2038 = property class="TabCtl (strict)"(reference=w2716, "Visible"=FALSE) -> ()  [unwired: 1 in, 2 out]
            n2039 = property class="TabCtl (strict)"(reference=w2709, "Visible"=FALSE) -> ()  [unwired: 1 in, 2 out]
            n2040 = property class="TabCtl (strict)"(reference=w2717, "Visible"=FALSE) -> ()  [unwired: 1 in, 2 out]
          }
          frame 8 {
            n2041 = control-ref of="PhaseB Experiment Option"() -> (w2794:refnum<vi>)
            n2042 = control-ref of="PhaseF Experiment Option"() -> (w2776:refnum<vi>)
            n2043 = control-ref of="PhaseA Experiment Option"() -> (w2796:refnum<vi>)
            n2044 = control-ref of="PhaseD Experiment Option"() -> (w2784:refnum<vi>)
            n2045 = control-ref of="PhaseC Experiment Option"() -> (w2785:refnum<vi>)
            n2046 = control-ref of="PhaseE Experiment Option"() -> (w2777:refnum<vi>)
            n2047 = property class="CmbBox"(reference=w2796, "Visible"=TRUE) -> ()  [unwired: 1 in, 2 out]
            n2048 = property class="CmbBox"(reference=w2794, "Visible"=TRUE) -> ()  [unwired: 1 in, 2 out]
            n2049 = property class="CmbBox"(reference=w2776, "Visible"=TRUE) -> ()  [unwired: 1 in, 2 out]
            n2050 = property class="CmbBox"(reference=w2784, "Visible"=TRUE) -> ()  [unwired: 1 in, 2 out]
            n2051 = property class="CmbBox"(reference=w2785, "Visible"=TRUE) -> ()  [unwired: 1 in, 2 out]
            n2052 = property class="CmbBox"(reference=w2777, "Visible"=TRUE) -> ()  [unwired: 1 in, 2 out]
            n2053 = control-ref of="Experiment Selection B"() -> (w2791:refnum<vi>)
            n2054 = control-ref of="Experiment Selection F"() -> (w2773:refnum<vi>)
            n2055 = control-ref of="Experiment Selection D"() -> (w2781:refnum<vi>)
            n2056 = control-ref of="Experiment Selection A"() -> (w2789:refnum<vi>)
            n2057 = control-ref of="Experiment Selection C"() -> (w2788:refnum<vi>)
            n2058 = control-ref of="Experiment Selection E"() -> (w2780:refnum<vi>)
            n2059 = property class="TabCtl (strict)"(reference=w2791, "Visible"=TRUE) -> ()  [unwired: 1 in, 2 out]
            n2060 = property class="TabCtl (strict)"(reference=w2789, "Visible"=TRUE) -> ()  [unwired: 1 in, 2 out]
            n2061 = property class="TabCtl (strict)"(reference=w2773, "Visible"=TRUE) -> ()  [unwired: 1 in, 2 out]
            n2062 = property class="TabCtl (strict)"(reference=w2781, "Visible"=TRUE) -> ()  [unwired: 1 in, 2 out]
            n2063 = property class="TabCtl (strict)"(reference=w2788, "Visible"=TRUE) -> ()  [unwired: 1 in, 2 out]
            n2064 = property class="TabCtl (strict)"(reference=w2780, "Visible"=TRUE) -> ()  [unwired: 1 in, 2 out]
            n2065 = control-ref of="PhaseH Experiment Option"() -> (w2751:refnum<vi>)
            n2066 = control-ref of="PhaseL Experiment Option"() -> (w2769:refnum<vi>)
            n2067 = control-ref of="PhaseG Experiment Option"() -> (w2749:refnum<vi>)
            n2068 = control-ref of="PhaseJ Experiment Option"() -> (w2761:refnum<vi>)
            n2069 = control-ref of="PhaseI Experiment Option"() -> (w2760:refnum<vi>)
            n2070 = control-ref of="PhaseK Experiment Option"() -> (w2768:refnum<vi>)
            n2071 = property class="CmbBox"(reference=w2749, "Visible"=TRUE) -> ()  [unwired: 1 in, 2 out]
            n2072 = property class="CmbBox"(reference=w2751, "Visible"=TRUE) -> ()  [unwired: 1 in, 2 out]
            n2073 = property class="CmbBox"(reference=w2769, "Visible"=FALSE) -> ()  [unwired: 1 in, 2 out]
            n2074 = property class="CmbBox"(reference=w2761, "Visible"=FALSE) -> ()  [unwired: 1 in, 2 out]
            n2075 = property class="CmbBox"(reference=w2760, "Visible"=FALSE) -> ()  [unwired: 1 in, 2 out]
            n2076 = property class="CmbBox"(reference=w2768, "Visible"=FALSE) -> ()  [unwired: 1 in, 2 out]
            n2077 = control-ref of="Experiment Selection H"() -> (w2754:refnum<vi>)
            n2078 = control-ref of="Experiment Selection L"() -> (w2772:refnum<vi>)
            n2079 = control-ref of="Experiment Selection J"() -> (w2764:refnum<vi>)
            n2080 = control-ref of="Experiment Selection G"() -> (w2756:refnum<vi>)
            n2081 = control-ref of="Experiment Selection I"() -> (w2757:refnum<vi>)
            n2082 = control-ref of="Experiment Selection K"() -> (w2765:refnum<vi>)
            n2083 = property class="TabCtl (strict)"(reference=w2754, "Visible"=TRUE) -> ()  [unwired: 1 in, 2 out]
            n2084 = property class="TabCtl (strict)"(reference=w2756, "Visible"=TRUE) -> ()  [unwired: 1 in, 2 out]
            n2085 = property class="TabCtl (strict)"(reference=w2772, "Visible"=FALSE) -> ()  [unwired: 1 in, 2 out]
            n2086 = property class="TabCtl (strict)"(reference=w2764, "Visible"=FALSE) -> ()  [unwired: 1 in, 2 out]
            n2087 = property class="TabCtl (strict)"(reference=w2757, "Visible"=FALSE) -> ()  [unwired: 1 in, 2 out]
            n2088 = property class="TabCtl (strict)"(reference=w2765, "Visible"=FALSE) -> ()  [unwired: 1 in, 2 out]
          }
          frame 9 {
            n2089 = control-ref of="PhaseB Experiment Option"() -> (w2842:refnum<vi>)
            n2090 = control-ref of="PhaseF Experiment Option"() -> (w2824:refnum<vi>)
            n2091 = control-ref of="PhaseA Experiment Option"() -> (w2844:refnum<vi>)
            n2092 = control-ref of="PhaseD Experiment Option"() -> (w2832:refnum<vi>)
            n2093 = control-ref of="PhaseC Experiment Option"() -> (w2833:refnum<vi>)
            n2094 = control-ref of="PhaseE Experiment Option"() -> (w2825:refnum<vi>)
            n2095 = property class="CmbBox"(reference=w2844, "Visible"=TRUE) -> ()  [unwired: 1 in, 2 out]
            n2096 = property class="CmbBox"(reference=w2842, "Visible"=TRUE) -> ()  [unwired: 1 in, 2 out]
            n2097 = property class="CmbBox"(reference=w2824, "Visible"=TRUE) -> ()  [unwired: 1 in, 2 out]
            n2098 = property class="CmbBox"(reference=w2832, "Visible"=TRUE) -> ()  [unwired: 1 in, 2 out]
            n2099 = property class="CmbBox"(reference=w2833, "Visible"=TRUE) -> ()  [unwired: 1 in, 2 out]
            n2100 = property class="CmbBox"(reference=w2825, "Visible"=TRUE) -> ()  [unwired: 1 in, 2 out]
            n2101 = control-ref of="Experiment Selection B"() -> (w2839:refnum<vi>)
            n2102 = control-ref of="Experiment Selection F"() -> (w2821:refnum<vi>)
            n2103 = control-ref of="Experiment Selection D"() -> (w2829:refnum<vi>)
            n2104 = control-ref of="Experiment Selection A"() -> (w2837:refnum<vi>)
            n2105 = control-ref of="Experiment Selection C"() -> (w2836:refnum<vi>)
            n2106 = control-ref of="Experiment Selection E"() -> (w2828:refnum<vi>)
            n2107 = property class="TabCtl (strict)"(reference=w2839, "Visible"=TRUE) -> ()  [unwired: 1 in, 2 out]
            n2108 = property class="TabCtl (strict)"(reference=w2837, "Visible"=TRUE) -> ()  [unwired: 1 in, 2 out]
            n2109 = property class="TabCtl (strict)"(reference=w2821, "Visible"=TRUE) -> ()  [unwired: 1 in, 2 out]
            n2110 = property class="TabCtl (strict)"(reference=w2829, "Visible"=TRUE) -> ()  [unwired: 1 in, 2 out]
            n2111 = property class="TabCtl (strict)"(reference=w2836, "Visible"=TRUE) -> ()  [unwired: 1 in, 2 out]
            n2112 = property class="TabCtl (strict)"(reference=w2828, "Visible"=TRUE) -> ()  [unwired: 1 in, 2 out]
            n2113 = control-ref of="PhaseH Experiment Option"() -> (w2799:refnum<vi>)
            n2114 = control-ref of="PhaseL Experiment Option"() -> (w2817:refnum<vi>)
            n2115 = control-ref of="PhaseG Experiment Option"() -> (w2797:refnum<vi>)
            n2116 = control-ref of="PhaseJ Experiment Option"() -> (w2809:refnum<vi>)
            n2117 = control-ref of="PhaseI Experiment Option"() -> (w2808:refnum<vi>)
            n2118 = control-ref of="PhaseK Experiment Option"() -> (w2816:refnum<vi>)
            n2119 = property class="CmbBox"(reference=w2797, "Visible"=TRUE) -> ()  [unwired: 1 in, 2 out]
            n2120 = property class="CmbBox"(reference=w2799, "Visible"=TRUE) -> ()  [unwired: 1 in, 2 out]
            n2121 = property class="CmbBox"(reference=w2817, "Visible"=FALSE) -> ()  [unwired: 1 in, 2 out]
            n2122 = property class="CmbBox"(reference=w2809, "Visible"=FALSE) -> ()  [unwired: 1 in, 2 out]
            n2123 = property class="CmbBox"(reference=w2808, "Visible"=TRUE) -> ()  [unwired: 1 in, 2 out]
            n2124 = property class="CmbBox"(reference=w2816, "Visible"=FALSE) -> ()  [unwired: 1 in, 2 out]
            n2125 = control-ref of="Experiment Selection H"() -> (w2802:refnum<vi>)
            n2126 = control-ref of="Experiment Selection L"() -> (w2820:refnum<vi>)
            n2127 = control-ref of="Experiment Selection J"() -> (w2812:refnum<vi>)
            n2128 = control-ref of="Experiment Selection G"() -> (w2804:refnum<vi>)
            n2129 = control-ref of="Experiment Selection I"() -> (w2805:refnum<vi>)
            n2130 = control-ref of="Experiment Selection K"() -> (w2813:refnum<vi>)
            n2131 = property class="TabCtl (strict)"(reference=w2802, "Visible"=TRUE) -> ()  [unwired: 1 in, 2 out]
            n2132 = property class="TabCtl (strict)"(reference=w2804, "Visible"=TRUE) -> ()  [unwired: 1 in, 2 out]
            n2133 = property class="TabCtl (strict)"(reference=w2820, "Visible"=FALSE) -> ()  [unwired: 1 in, 2 out]
            n2134 = property class="TabCtl (strict)"(reference=w2812, "Visible"=FALSE) -> ()  [unwired: 1 in, 2 out]
            n2135 = property class="TabCtl (strict)"(reference=w2805, "Visible"=TRUE) -> ()  [unwired: 1 in, 2 out]
            n2136 = property class="TabCtl (strict)"(reference=w2813, "Visible"=FALSE) -> ()  [unwired: 1 in, 2 out]
          }
          frame 10 {
            n2137 = control-ref of="PhaseB Experiment Option"() -> (w2890:refnum<vi>)
            n2138 = control-ref of="PhaseF Experiment Option"() -> (w2872:refnum<vi>)
            n2139 = control-ref of="PhaseA Experiment Option"() -> (w2892:refnum<vi>)
            n2140 = control-ref of="PhaseD Experiment Option"() -> (w2880:refnum<vi>)